vi "15-12-13 UHR-Fleezers Control (host) - 15.2.1UCB Darwin.vi"() -> ()   [LabVIEW 2014] (continued)
            n3419 = flat-sequence {
              frame #0 {
                # "stop only if saving"
                n3420 = local read "Saving..."() -> (w4631:bool)
                n3421 = And(x=w4631, y="TA Cancel Save?") -> (x .and. y?=w4630:bool)
                n3422 = local write "Stop Saving"(w4630) -> ()
              }
              frame #1 {
                n3423 = case shown="True" "TA Green Off?" {
                  frame False {
                  }
                  frame True {
                    w4634 = FALSE ("Fl. Triggered...")
                    n3424 = local write "Fl. Triggered..."(w4634) -> ()
                    n3425 = property on="Green Laser ON" class="Bool (strict)"("Val(Sgnl)"=w4634) -> ()  [unwired: 2 in, 2 out]
                  }
                }
              }
            }
            n3426 = local read "Time tether formed"() -> (w4625:timestamp)
            n3427 = Get Date/Time In Seconds() -> (seconds since 1Jan1904=w4626:timestamp)
            n3428 = Subtract(x=w4626, y=w4625) -> (x-y=w4624:dbl)
            n3429 = Number To Decimal String(number=w4624) -> (decimal integer string=w4621:string)  [unwired: 1 out]
            n3430 = local read "Messages"() -> (w4628:string)
            n3431 = call <vilib>:"Beep.vi"() -> ()  [unwired: 3 in, 9 out]
            n3432 = Concatenate Strings("Lost tether (" ("Message to add"), w4621, " s)." ("string")) -> (w4623:string)
            n3433 = local write "Tether"(FALSE ("Tether")) -> ()
            n3434 = call "Update messages.vi"("Message to add"=w4623, "Old message string"=w4628) -> ("New message string"=w4627:string)
            n3435 = local write "Messages"(w4627) -> ()
            n3436 = property on="Fl. Triggered..." class="Bool (strict)"("Val(Sgnl)"=w4619) -> ()  [unwired: 2 in, 2 out]
            n3437 = local write "Dip for Protein"(w4619) -> ()
            n3438 = property on="Trap Pos. FB ON" class="Bool (strict)"("Val(Sgnl)"=w4619) -> ()  [unwired: 2 in, 2 out]
            n3439 = property on="Trap Trig. Fl." class="Bool (strict)"("Val(Sgnl)"=w4619) -> ()  [unwired: 2 in, 2 out]
          }
        }
      }
    }
    n3440 = case "For triggering actions based on the trap position (e.g., turning the excitation laser on if trap under feedback moves so far)" shown="True" "Trap Trig. Fl." {
      tunnel: w4110 -> [_ w4507]
      tunnel: w4123 -> [_ w4506]
      tunnel: ["" ("t") w4505] -> w4131
      tunnel: w4115 -> [_ w4504]
      tunnel: [0 ("t") w4503] -> w4128
      tunnel: w4127 -> [_ w4502]
      tunnel: w4102 -> [_ w4501]
      tunnel: w4101 -> [_ w4500]
      frame False {
      }
      frame True {
        n3441 = case shown="\"Wait for trigger\"" w4506 {
          tunnel: w4507 -> [w4524 _ _ w4572]
          tunnel: [w4521 w4553 "" ("t") w4575] -> w4505
          tunnel: w4504 -> [_ _ _ w4563]
          tunnel: [w4520 w4550 0 ("t") w4564] -> w4503
          tunnel: w4502 -> [_ w4552 _ w4570]
          tunnel: w4501 -> [w4509 w4547 _ w4566]
          tunnel: w4500 -> [w4508 w4546 _ w4565]
          frame "Wait for trigger" {
            n3442 = local read "Trap Trig. (FPGA)"() -> (w4512:bool)
            n3443 = Subtract(x=w4524, y="Mean T1 Position\nto compare (nm)") -> (x-y=w4517:dbl[])
            n3444 = call <vilib>:"Std Deviation and Variance.vi"("X"=w4517) -> ("mean"=→"mean":dbl, "standard deviation"=→"standard\ndeviation":dbl)  [unwired: 1 in, 1 out]
            n3445 = Array Max & Min(array=w4517) -> (max value=→"max value":dbl, min value=→"min value":dbl)  [unwired: 2 out]
            n3446 = Greater?(x=w4517, y="Threshold (nm)") -> (0:w4527:bool[])
            n3447 = case shown="True" w4512 {
              tunnel: w4509 -> [_ w4533]
              tunnel: w4508 -> [_ w4532]
              tunnel: [FALSE ("TTrig?") w4531] -> w4515
              frame False {
              }
              frame True {
                n3448 = xnode "Read/Write Control"("FPGA VI Reference In"=w4533, "error in"=w4532) -> ("TTrig?"=w4531:bool)  [unwired: 2 out]
              }
            }
            n3449 = Or Array Elements(Boolean array=w4527) -> (logical OR=w4514:bool)
            n3450 = Select(t=w4515, s=w4512, f=w4514) -> (s? t:f=w4513:bool)
            n3451 = Not(x=w4512) -> (.not. x?=w4511:bool)
            n3452 = And(x=w4513, y=w4511) -> (x .and. y?=w4510:bool)
            n3453 = Select(t="Triggered", s=w4513, f="Wait for trigger") -> (s? t:f=w4521:string)
            n3454 = case shown="True" w4513 {
              tunnel: [0 0] -> w4520
              tunnel: w4509 -> [_ w4538]
              tunnel: w4508 -> [_ w4537]
              frame False {
                "Waiting" <- TRUE ("Waiting")
              }
              frame True {
                n3455 = xnode "Read/Write Control"("FPGA VI Reference In"=w4538, "error in"=w4537, "TTrig?"=FALSE) -> ()  [unwired: 2 out]
                n3456 = local read "Messages"() -> (w4541:string)
                n3457 = call <vilib>:"Beep.vi"() -> ()  [unwired: 12 in]
                n3458 = call "Update messages.vi"("Message to add"="Unwinding trigger.", "Old message string"=w4541) -> ("New message string"=w4542:string)
                n3459 = local write "Messages"(w4542) -> ()
                n3460 = local write "Waiting"(FALSE ("Waiting")) -> ()
                "Triggered" <- TRUE ("Triggered")
              }
            }
            n3461 = case "Only need to turn on laser if host triggered" shown="True" w4510 {
              frame False {
              }
              frame True {
                n3462 = property on="Green Laser ON" class="Bool (strict)"("Val(Sgnl)"=TRUE ("Value (Signaling)")) -> ()  [unwired: 2 in, 2 out]
              }
            }
          }
          frame "Triggered" {
            n3463 = local read "Trap Trig. (FPGA)"() -> (w4549:bool)
            n3464 = Increment(x=w4552) -> (x+1=w4550:i32)
            n3465 = Greater Or Equal?(x=w4550, y="Fl. ON time (n)") -> (x >= y?=w4548:bool)
            n3466 = Select(t="Wait for trigger", s=w4548, f="Triggered" ("t")) -> (s? t:f=w4553:string)
            n3467 = And(x=w4548, y=w4549) -> (x .and. y?=w4545:bool)
            n3468 = case shown="True" w4545 {
              tunnel: w4547 -> [_ w4557]
              tunnel: w4546 -> [_ w4556]
              frame False {
              }
              frame True {
                n3469 = xnode "Read/Write Control"("FPGA VI Reference In"=w4557, "error in"=w4556, "FPGA Trap Trig"=TRUE) -> ()  [unwired: 2 out]
              }
            }
            n3470 = case shown="True" w4548 {
              frame False {
              }
              frame True {
                w4559 = FALSE ("Value (Signaling)")
                n3471 = local write "Triggered"(w4559) -> ()
                n3472 = local write "Waiting"(TRUE ("Waiting")) -> ()
                n3473 = property on="Green Laser ON" class="Bool (strict)"("Val(Sgnl)"=w4559) -> ()  [unwired: 2 in, 2 out]
              }
            }
          }
          frame "Do nothing" {
          }
          frame "Initialize", Default {
            n3474 = Increment(x=w4570) -> (x+1=w4574:i32)
            n3475 = Select(t=1, s=w4563, f=w4574) -> (s? t:f=w4564:i32)
            n3476 = feedback #28(w4572) -> (w4578:dbl[])
            n3477 = Build Array (concatenate)(w4572, w4578) -> (w4571:dbl[])
            n3478 = Greater Or Equal?(x=w4564, y="Wait to get offset (n)") -> (x >= y?=w4567:bool)
            n3479 = Select(t=w4572, s=w4563, f=w4571) -> (s? t:f=w4573:dbl[])
            n3480 = feedback-in #28(w4573) -> ()
            n3481 = call-poly <vilib>:"Mean.vi"("X"=w4573) -> ("mean"=w4568:dbl)  [unwired: 1 out]
            n3482 = local write "Mean T1 Position\nto compare (nm)"(w4568) -> ()
            n3483 = case shown="True" w4563 {
              tunnel: w4566 -> [_ w4584]
              tunnel: w4565 -> [_ w4583]
              frame False {
              }
              frame True {
                w4580 = FALSE ("FPGA Trap Trig")
                n3484 = xnode "Read/Write Control"("FPGA VI Reference In"=w4584, "error in"=w4583, "FPGA Trap Trig"=w4580) -> ("FPGA VI Reference Out"=w4582:T24, "error out"=w4581:errorcluster)
                n3485 = xnode "Read/Write Control"("FPGA VI Reference In"=w4582, "error in"=w4581, "TTrig?"=w4580) -> ()  [unwired: 2 out]
              }
            }
            n3486 = Select(t="Wait for trigger", s=w4567, f="Initialize") -> (s? t:f=w4575:string)
            n3487 = case shown="True" w4567 {
              tunnel: w4568 -> [_ w4587]
              tunnel: w4566 -> [_ w4596]
              tunnel: w4565 -> [_ w4595]
              frame False {
                n3488 = local write "Waiting"(FALSE ("Waiting")) -> ()
                "Initializing" <- TRUE ("Initializing")
              }
              frame True {
                n3489 = local read "Threshold (nm)"() -> (w4599:dbl)
                n3490 = local read "AOM X Cal (nm/MHz)"() -> (w4598:dbl)
                n3491 = Add(x=w4587, y=w4599) -> (x+y=w4600:dbl)
                n3492 = Divide(x=w4600, y=w4598) -> (x/y=w4597:dbl)
                n3493 = call "IR AOM freq to word.vi"("Frequency In (MHz)"=w4597) -> ("Frequency Word Out (double)"=w4594:dbl)
                n3494 = local write "Initializing"(FALSE ("Initializing")) -> ()
                n3495 = local write "Waiting"(TRUE ("Waiting")) -> ()
                n3496 = To Quad Integer(1:w4594) -> (0:w4593:i64)
                n3497 = xnode "Read/Write Control"("FPGA VI Reference In"=w4596, "error in"=w4595, "FPGA TTrig Thresh"=w4593) -> ("FPGA VI Reference Out"=w4590:T24, "error out"=w4589:errorcluster)
                n3498 = xnode "Read/Write Control"("FPGA VI Reference In"=w4590, "error in"=w4589, "FPGA Trap Trig"=TRUE) -> ()  [unwired: 2 out]
              }
            }
          }
        }
      }
    }
    n3499 = feedback-in #26(w4131) -> ()
    n3500 = feedback-in #27(w4128) -> ()
    n3501 = xnode ("Read/Write Control")("FPGA VI Reference In"=w4270, "error in"=w4269) -> ("FPGA VI Reference Out"=w4113:T24, "error out"=w4112:errorcluster, "AI2 Y Sum Set 1"=w4342:i16, "AI2 Y Sum Set 2"=w4341:i16, "AI1 X Set 1"=w4177:fxp<+/-,16,1>, "AI1 X Set 2"=w4176:fxp<+/-,16,1>, "Trap Pos FB Int Signal"=→"Trap Pos FB Int Signal":fxp<+/-,24,9>, "Trap Pos FB Int-Norm Signal"=→"Trap Pos FB Int-Norm Signal":fxp<+/-,16,1>, "Trap Pos FB Action"=w4170:i64, "Scanning"=→"AOD Scanning":bool, "Scan I"=→"AOD Scan I":u64, "Scanning MCL"=w4344:bool, "Scan I (MCL)"=→"MCL Scan I":u64, "Green FB Sum"=w4286:i16, "Trap Pos FB Action"=w4100:i64, "TTrig Fin Thresh"=w4096:i64, "Red FB Intensity"=w4080:i16, "Blue Intensity"=w4075:i16)
    "MCL Scanning" <- w4344
    "Trap Pos FB Action" <- w4170
    n3502 = Divide(x=w4080, y=3276.7) -> (x/y=w4079:dbl)
    "Red laser intensity (V)" <- w4079
    n3503 = Divide(x=w4075, y=3276.7) -> (x/y=w4074:dbl)
    "Blue laser intensity (V)" <- w4074
    n3504 = Divide(x=w4286, y=3276.7) -> (x/y=w4078:dbl)
    "Green laser intensity (V)" <- w4078
    n3505 = local read "FB Trig Integrate"() -> (w4094:u32)
    n3506 = Divide(x=w4100, y=w4094) -> (x/y=w4093:dbl)
    "TTrig Sig (Int)" <- w4093
    n3507 = Bundle(w4078, w4079, w4074) -> (→"Fluorescence laser intensities plot":cluster{dbl, dbl, dbl})  [unwired: 1 in]
    n3508 = Divide(x=w4096, y=w4094) -> (x/y=w4091:dbl)
    "TTrig Fin Thresh (Int)" <- w4091
    n3509 = local read "AOM X Cal (nm/MHz)"() -> (w4099:dbl)
    n3510 = local read "AI2 (V)"() -> (w4343:cluster{"Set 1":dbl, "Set 2":dbl})
    n3511 = Bundle By Name(cluster=w4343, "Set 1"=w4342, "Set 2"=w4341) -> (w4339:cluster{"Set 1":dbl, "Set 2":dbl})
    n3512 = Divide(x=w4170, y=327.67) -> (x/y=→"Action (%)":dbl)
    n3513 = local read "Trap X (AI1)"() -> (w4190:T12)
    n3514 = call "IR AOM word double to freq.vi"("Frequency Word In (double)"=w4091) -> ("Frequency Out (MHz)"=w4090:dbl)
    n3515 = call "IR AOM word double to freq.vi"("Frequency Word In (double)"=w4093) -> ("Frequency Out (MHz)"=w4092:dbl)
    n3516 = Divide(x=w4339, y=3276.7) -> (x/y=w4338:cluster{"Set 1":dbl, "Set 2":dbl})
    n3517 = Multiply(x=w4092, y=w4099) -> (x*y=w4098:dbl)
    "TTrig Sig (nm)" <- w4098
    n3518 = Multiply(x=w4090, y=w4099) -> (x*y=w4097:dbl)
    "TTrig Fin Thresh (nm)" <- w4097
    n3519 = local write "AI2 (V)"(w4338) -> ()
    n3520 = Bundle(cluster=w4190, "Trap 1"=w4177, "Trap 2"=w4176) -> (→"Trap X (AI1)":T12)
    n3521 = Bundle(w4098, w4097) -> (→"TTrig":cluster{dbl, dbl})  [unwired: 1 in]
    n3522 = flat-sequence "To save data" {
      tunnel: [w5479] -> w4362
      tunnel: [w5480] -> w4361
      tunnel: w4315 -> [w5473]
      tunnel: w4118 -> [w5477]
      tunnel: ["Save Calibration"] -> w4335
      tunnel: w4332 -> [w5476]
      tunnel: [w5469] -> w4331
      tunnel: [w5466] -> w4330
      tunnel: [w5463] -> w4329
      tunnel: w4314 -> [w5465]
      tunnel: w4254 -> [w5459]
      tunnel: [w5459] -> w4253
      tunnel: [w5451] -> w4227
      tunnel: [w5454] -> w4158
      tunnel: [w5453] -> w4157
      tunnel: [w5447] -> w4008
      tunnel: w4362 -> [w5757]
      tunnel: w4361 -> [w5756]
      tunnel: w4159 -> [w5755]
      tunnel: w4335 -> [w5754]
      tunnel: w4331 -> [w5752]
      tunnel: w4330 -> [w5751]
      tunnel: w4329 -> [w5750]
      tunnel: w4235 -> [w5749]
      tunnel: w4262 -> [w5748]
      tunnel: w4253 -> [w5747]
      tunnel: w4227 -> [w5746]
      tunnel: w4015 -> [w5745]
      tunnel: w4060 -> [w5744]
      tunnel: w4158 -> [w5743]
      tunnel: w4157 -> [w5742]
      tunnel: w4156 -> [w5741]
      tunnel: w4082 -> [w5740]
      tunnel: w4006 -> [w5739]
      tunnel: w4008 -> [w5738]
      frame #0 {
        n3523 = Or(x="Start Saving", y="Start saving data + video") -> (x .or. y?=w5451:bool)
        n3524 = case shown="True" "Start saving data + video" {
          frame False {
          }
          frame True {
            n3525 = stacked-sequence {
              frame #0 {
                n3526 = local write "New Video File"(TRUE ("New Video File")) -> ()
              }
              frame #1 {
                n3527 = local write "Save Video"(TRUE ("Save Video")) -> ()
              }
            }
          }
        }
        n3528 = Or(x="Save N Sets", y=w5451) -> (x .or. y?=w5460:bool)
        n3529 = To Double Precision Float(number=w5476) -> (double precision float=w5470:dbl)
        n3530 = Build Array(w5460, "Save Calibration", w5473, w5465) -> (w5475:bool[])
        n3531 = Compound Arithmetic op=OR("Save Calibration", w5473, w5460, w5465) -> (w5478:bool)
        n3532 = Boolean Array To Number(Boolean array=w5475) -> (number=w5472:u32)
        n3533 = feedback #29(FALSE ("Save APD Data\nwith Trap Data")) -> (w5455:bool)
        n3534 = feedback #30(refnum<k0> refnum) -> (w5481:refnum<file>)
        n3535 = feedback #31(FALSE ("Save APD Data\nwith Trap Data")) -> (w5464:bool)
        n3536 = feedback #32(0) -> (w5483:i32)
        n3537 = feedback #33() -> (w5471:u32)  [unwired: 1 out]
        n3538 = feedback #34(refnum<k0> refnum) -> (w5448:refnum<file>)
        n3539 = feedback #35(refnum<k0> refnum) -> (w5457:refnum<file>)
        n3540 = feedback #36(refnum<k0> refnum) -> (w5467:refnum<file>)
        n3541 = case shown="True" w5478 {
          tunnel: [w5493 1] -> w5479
          tunnel: w5483 -> [w5495 _]
          tunnel: [w5494 w5528] -> w5480
          tunnel: w5481 -> [w5494 _]
          tunnel: w5477 -> [_ w5546]
          tunnel: w5470 -> [_ w5544]
          tunnel: w5472 -> [_ w5547]
          tunnel: [w5492 w5527] -> w5469
          tunnel: w5471 -> [w5492 _]
          tunnel: [w5491 w5525] -> w5466
          tunnel: w5467 -> [w5491 _]
          tunnel: [w5490 w5524] -> w5463
          tunnel: w5464 -> [w5490 _]
          tunnel: w5451 -> [_ w5522]
          tunnel: w5459 -> [_ w5521]
          tunnel: [w5489 w5513] -> w5453
          tunnel: w5457 -> [w5489 _]
          tunnel: [w5488 w5512] -> w5454
          tunnel: w5455 -> [w5488 _]
          tunnel: [w5487 w5496] -> w5447
          tunnel: w5448 -> [w5487 _]
          frame False {
            n3542 = Increment(x=w5495) -> (x+1=w5493:i32)
          }
          frame True {
            w5518 = FALSE ("Start Saving")
            w5523 = 9.0  # File Version
            w5530 = FALSE ("prepend array or string size? (T)")
            w5529 = T32."big-endian, network order" ("byte order (0:big-endian, network order)")
            # "Save trap position\ndata"
            n3543 = local read "BD 1 Frequency 1 (MHz)"() -> (w5543:dbl)
            n3544 = local read "BD 2 Frequency 1 (MHz)"() -> (w5542:dbl)
            n3545 = local read "BD 1 Frequency 2 (MHz)"() -> (w5541:dbl)
            n3546 = local read "BD 2 Frequency 2 (MHz)"() -> (w5540:dbl)
            n3547 = local read "BD 1 Frequency 3 (MHz)"() -> (w5539:dbl)
            n3548 = local read "BD 2 Frequency 3 (MHz)"() -> (w5538:dbl)
            n3549 = Array Size(array=w5521) -> (size(s)=w5520:i32)
            n3550 = To Double Precision Float(number=w5520) -> (double precision float=w5519:dbl)
            n3551 = local write "Save Calibration"(w5518) -> ()
            n3552 = local write "Start Saving"(w5518) -> ()
            n3553 = Build Array("Save APD Data\nwith Trap Data", "Save Trap Pos. Data") -> (w5515:bool[])
            n3554 = Boolean Array To Number(Boolean array=w5515) -> (number=w5514:u32)
            n3555 = Build Array(w5543, w5542, w5541, w5540, w5539, w5538) -> (w5537:dbl[])
            n3556 = case shown="2" w5547 {
              tunnel: w5546 -> [w5635 w5662 w5678 w5716]
              tunnel: w5519 -> [w5640 w5669 w5698 w5735]
              tunnel: w5544 -> [w5639 w5668 w5697 w5734]
              tunnel: [w5636 w5664 w5689 w5726] -> w5535
              tunnel: [w5627 "Cal sets to save" w5679 w5717] -> w5527
              tunnel: w5537 -> [w5637 w5665 w5691 w5728]
              tunnel: "Save APD Data\nwith Trap Data" -> [w5634 w5651 w5675 w5714]
              tunnel: [w5634 w5649 w5675 w5714] -> w5524
              tunnel: w5523 -> [w5630 w5658 w5673 w5712]
              tunnel: w5522 -> [w5629 _ _ _]
              tunnel: [w5620 w5657 w5672 w5702] -> w5512
              tunnel: "Save Trap Pos. Data" -> [w5620 w5656 w5672 w5702]
              tunnel: w5514 -> [w5619 w5655 w5671 w5701]
              frame 1, Default {
                # "timeseries"
                n3557 = case shown="False" "Profile" {
                  tunnel: [w5643 w5647] -> w5624
                  tunnel: [w5643 w5646] -> w5623
                  tunnel: [w5643 w5645] -> w5622
                  tunnel: [w5643 w5644] -> w5621
                  frame False {
                    w5643 = 0.0 ("f")
                  }
                  frame True {
                    n3558 = local read "Current Position"() -> (w5648:cluster{dbl, dbl, dbl})
                    n3559 = local read "Y change (mm)"() -> (w5644:dbl)
                    n3560 = Unbundle(w5648) -> (w5647:dbl, w5646:dbl, w5645:dbl)
                  }
                }
                n3561 = local read "Save ave N"() -> (w5642:dbl)
                n3562 = Multiply(x=w5642, y=w5635) -> (x*y=w5641:dbl)
                n3563 = To Double Precision Float(number=w5619) -> (double precision float=w5633:dbl)
                n3564 = Build Array(w5630, w5635, w5641, w5640, w5639, 0.0 ("f")) -> (w5638:dbl[])
                n3565 = Build Array(w5633, w5624, w5623, w5622, w5621) -> (w5631:dbl[])
                n3566 = Select(t=u32 4000000000, s=w5629, f="N sets to save") -> (s? t:f=w5627:u32)
                n3567 = Build Array (concatenate)(w5638, w5637, w5631) -> (w5636:dbl[])
              }
              frame 2 {
                w5660 = 0.0 ("f")
                w5650 = FALSE ("Save APD Data\nwith Trap Data")
                # "For diagnostics save trap position\ndata during cal"
                # "calibration"
                n3568 = Boolean To (0,1)(Boolean=w5650) -> (0, 1=w5654:i16)
                n3569 = Select(t=w5651, s="Save trap pos with cal", f=w5650) -> (s? t:f=w5649:bool)
                n3570 = Select(t=w5656, s="Save trap pos with cal", f=w5650) -> (s? t:f=w5657:bool)
                n3571 = Select(t=w5655, s="Save trap pos with cal", f=w5654) -> (s? t:f=w5653:u32)
                n3572 = To Double Precision Float(number=w5653) -> (double precision float=w5661:dbl)
                n3573 = Build Array(w5658, w5662, w5662, w5669, w5668, 1.0 ("t")) -> (w5666:dbl[])
                n3574 = Build Array(w5661, w5660, w5660, w5660, w5660) -> (w5659:dbl[])
                n3575 = Build Array (concatenate)(w5666, w5665, w5659) -> (w5664:dbl[])
                "Calibrating Trap..." <- TRUE ("Calibrating...")
              }
              frame 4 {
                w5676 = 0.0 ("f")
                # "scan dir (x/y = 0/1)"
                # "cycles/step"
                # "n scans (f/b)"
                # "steps"
                # "freq. range"
                # "AOD raster scan"
                n3576 = local read "Number of F/B Scans (AOD)"() -> (w5683:u16)
                n3577 = local read "Cycles/step (AOD)"() -> (w5685:u64)
                n3578 = local read "Scan Range (MHz)"() -> (w5688:dbl)
                n3579 = local read "Scan steps (AOD)"() -> (w5687:u64)
                n3580 = local read "Scan BD"() -> (w5695:bool)
                n3581 = local read "Save ave N"() -> (w5700:dbl)
                n3582 = Boolean To (0,1)(Boolean=w5695) -> (0, 1=w5694:i16)
                n3583 = To Double Precision Float(number=w5683) -> (double precision float=w5682:dbl)
                n3584 = To Double Precision Float(number=w5687) -> (double precision float=w5686:dbl)
                n3585 = To Double Precision Float(number=w5685) -> (double precision float=w5684:dbl)
                n3586 = To Double Precision Float(number=w5694) -> (double precision float=w5693:dbl)
                n3587 = Multiply(x=w5700, y=w5678) -> (x*y=w5699:dbl)
                n3588 = To Double Precision Float(number=w5671) -> (double precision float=w5677:dbl)
                n3589 = Build Array(w5677, w5676, w5676, w5676, w5676) -> (w5674:dbl[])
                n3590 = local read "N sets should be saved"() -> (w5680:dbl)
                n3591 = Build Array(w5693, w5688, w5686, w5684, w5682) -> (w5690:dbl[])
                n3592 = Build Array(w5673, w5678, w5699, w5698, w5697, 2.0 ("t")) -> (w5692:dbl[])
                n3593 = Round Toward +Infinity(x=w5680) -> (ceil(x): smallest int >= x=w5681:dbl)
                n3594 = Build Array (concatenate)(w5692, w5691, w5674, w5690) -> (w5689:dbl[])
                n3595 = To Unsigned Long Integer(number=w5681) -> (unsigned 32bit integer=w5679:u32)
              }
              frame 8 {
                w5709 = 0.0 ("f")
                # "MCL raster scan"
                n3596 = local read "Number of scans (MCL)"() -> (w5704:u64)
                n3597 = local read "Scan lines (y)"() -> (w5703:u64)
                n3598 = local read "2D or 1D Scan"() -> (w5706:bool)
                n3599 = local read "Scan Range (V)\n(of steps)"() -> (w5725:dbl)
                n3600 = local read "Fast Scan Dir"() -> (w5732:bool)
                n3601 = local read "Cycles/step (MCL)"() -> (w5722:u64)
                n3602 = local read "Scan steps (MCL)"() -> (w5724:u64)
                n3603 = Select(t=w5703, s=w5706, f=w5704) -> (s? t:f=w5705:u64)
                n3604 = Boolean To (0,1)(Boolean=w5706) -> (0, 1=w5708:i16)
                n3605 = local read "Save ave N"() -> (w5737:dbl)
                n3606 = local read "Initial X"() -> (w5711:dbl)
                n3607 = local read "Initial Y"() -> (w5710:dbl)
                n3608 = To Double Precision Float(number=w5708) -> (double precision float=w5707:dbl)
                n3609 = Boolean To (0,1)(Boolean=w5732) -> (0, 1=w5731:i16)
                n3610 = To Double Precision Float(number=w5705) -> (double precision float=w5720:dbl)
                n3611 = To Double Precision Float(number=w5724) -> (double precision float=w5723:dbl)
                n3612 = To Double Precision Float(number=w5722) -> (double precision float=w5721:dbl)
                n3613 = To Double Precision Float(number=w5731) -> (double precision float=w5730:dbl)
                n3614 = Multiply(x=w5737, y=w5716) -> (x*y=w5736:dbl)
                n3615 = To Double Precision Float(number=w5701) -> (double precision float=w5715:dbl)
                n3616 = local read "N sets should be saved (MCL)"() -> (w5718:dbl)
                n3617 = Build Array(w5715, w5707, w5709, w5709, w5709) -> (w5713:dbl[])
                n3618 = Build Array(w5730, w5725, w5723, w5721, w5720, w5711, w5710) -> (w5727:dbl[])
                n3619 = Build Array(w5712, w5716, w5736, w5735, w5734, 3.0 ("t")) -> (w5729:dbl[])
                n3620 = Round Toward +Infinity(x=w5718) -> (ceil(x): smallest int >= x=w5719:dbl)
                n3621 = Build Array (concatenate)(w5729, w5728, w5713, w5727) -> (w5726:dbl[])
                n3622 = To Unsigned Long Integer(number=w5719) -> (unsigned 32bit integer=w5717:u32)
              }
            }
            n3623 = local read "Index"() -> (w5552:dbl)
            n3624 = call "Create new save file.vi"("Insert"="", "Ext"=".dat", "Index In"=w5552) -> ("Path Out"=w5498:path, "Index Out"=w5526:dbl)
            n3625 = local write "Save file name"(w5498) -> ()
            n3626 = local write "Index"(w5526) -> ()
            n3627 = local write "Save index"(w5526) -> ()
            n3628 = case shown="True" "Save Event Log?" {
              tunnel: w5498 -> [_ w5560]
              tunnel: [refnum<k0> refnum w5559] -> w5496
              frame False {
              }
              frame True {
                (unwired) FALSE ("prepend array or string size? (T)")
                n3629 = Path To String(path=w5560) -> (string=w5571:string)
                n3630 = String Length(string=w5571) -> (length=w5570:i32)
                n3631 = Subtract(x=w5570, y=4) -> (x-y=w5568:i32)
                n3632 = String Subset(string=w5571, length (rest)=w5568) -> (substring=w5567:string)  [unwired: 1 out]
                n3633 = Concatenate Strings(w5567, "_log.txt" ("string")) -> (w5565:string)
                n3634 = String To Path(string=w5565) -> (path=w5561:path)
                n3635 = Open/Create/Replace File(file path (use dialog)=w5561, operation (0:open)=T33."create", access (0:read/write)=enum16{"read/write", "read-only", "write-only"}."write-only") -> (refnum out=w5562:refnum<file>)  [unwired: 1 in, 4 out]
                n3636 = Deny Access(7:w5562) -> (3:w5559:refnum<file>)  [unwired: 1 in, 2 out]
                n3637 = call "write to event log.vi"("log file ref"=w5559, "time"=0.0, "input string"="start log") -> ()  [unwired: 8 in]
              }
            }
            "log file ref" <- w5496
            n3638 = Array Size(array=w5535) -> (size(s)=w5536:i32)
            n3639 = Open/Create/Replace File(file path (use dialog)=w5498, operation (0:open)=T33."create", access (0:read/write)=enum16{"read/write", "read-only", "write-only"}."write-only") -> (refnum out=w5549:refnum<file>)  [unwired: 1 in, 4 out]
            n3640 = local write "Saving..."(TRUE ("Saving...")) -> ()
            n3641 = To Double Precision Float(number=w5536) -> (double precision float=w5534:dbl)
            n3642 = String Length(string="Comment (data description)") -> (length=w5533:i32)
            n3643 = To Double Precision Float(number=w5533) -> (double precision float=w5532:dbl)
            n3644 = Deny Access(7:w5549) -> (3:w5548:refnum<file>)  [unwired: 1 in, 2 out]
            n3645 = Build Array (concatenate)(w5534, w5535, w5532) -> (w5508:dbl[])
            n3646 = case "If fluorescence data to be saved" shown="True" w5524 {
              tunnel: w5498 -> [_ w5618]
              tunnel: [refnum<k0> refnum w5598] -> w5525
              frame False {
              }
              frame True {
                w5597 = 0.0
                n3647 = local read "APD Integration Time (s)"() -> (w5603:dbl)
                n3648 = local read "N APD Samp/step"() -> (w5596:dbl)
                n3649 = local read "Number of APDs"() -> (w5595:u8)
                n3650 = Path To String(path=w5618) -> (string=w5617:string)
                n3651 = String Length(string=w5617) -> (length=w5616:i32)
                n3652 = Subtract(x=w5616, y=4) -> (x-y=w5614:i32)
                n3653 = String Subset(string=w5617, length (rest)=w5614) -> (substring=w5613:string)  [unwired: 1 out]
                n3654 = Build Array(w5603, w5596, w5595, w5597, w5597, w5597, w5597, w5597) -> (w5600:dbl[])
                n3655 = Concatenate Strings(w5613, "_fl.dat" ("string")) -> (w5611:string)
                n3656 = Array Size(array=w5600) -> (size(s)=w5602:i32)
                n3657 = String To Path(string=w5611) -> (path=w5607:path)
                n3658 = Open/Create/Replace File(file path (use dialog)=w5607, operation (0:open)=T33."create", access (0:read/write)=enum16{"read/write", "read-only", "write-only"}."write-only") -> (refnum out=w5608:refnum<file>)  [unwired: 1 in, 4 out]
                n3659 = Deny Access(7:w5608) -> (3:w5604:refnum<file>)  [unwired: 1 in, 2 out]
                n3660 = To Double Precision Float(number=w5602) -> (double precision float=w5601:dbl)
                n3661 = Build Array (concatenate)(w5601, w5600) -> (w5599:dbl[])
                n3662 = Write to Binary File(file (use dialog)=w5604, data=w5599, 5:FALSE ("prepend array or string size? (T)"), 9:T32."big-endian, network order" ("byte order (0:big-endian, network order)")) -> (refnum out=w5598:refnum<file>)  [unwired: 1 in, 3 out]
              }
            }
            n3663 = case shown="True" w5512 {
              tunnel: w5498 -> [_ w5579]
              tunnel: [refnum<k0> refnum w5578] -> w5513
              frame False {
              }
              frame True {
                w5574 = 0.0 ("element")
                n3664 = Path To String(path=w5579) -> (string=w5593:string)
                n3665 = Build Array(w5574, w5574, w5574, w5574, w5574, w5574, w5574, w5574) -> (w5575:dbl[])
                n3666 = String Length(string=w5593) -> (length=w5592:i32)
                n3667 = Subtract(x=w5592, y=4) -> (x-y=w5590:i32)
                n3668 = Array Size(array=w5575) -> (size(s)=w5577:i32)
                n3669 = String Subset(string=w5593, length (rest)=w5590) -> (substring=w5589:string)  [unwired: 1 out]
                n3670 = To Double Precision Float(number=w5577) -> (double precision float=w5576:dbl)
                n3671 = Concatenate Strings(w5589, "_pos.dat" ("string")) -> (w5587:string)
                n3672 = Build Array (concatenate)(w5576, w5575) -> (w5573:dbl[])
                n3673 = String To Path(string=w5587) -> (path=w5583:path)
                n3674 = Open/Create/Replace File(file path (use dialog)=w5583, operation (0:open)=T33."create", access (0:read/write)=enum16{"read/write", "read-only", "write-only"}."write-only") -> (refnum out=w5584:refnum<file>)  [unwired: 1 in, 4 out]
                n3675 = Deny Access(7:w5584) -> (3:w5580:refnum<file>)  [unwired: 1 in, 2 out]
                n3676 = Write to Binary File(file (use dialog)=w5580, data=w5573, 5:FALSE ("prepend array or string size? (T)"), 9:T32."big-endian, network order" ("byte order (0:big-endian, network order)")) -> (refnum out=w5578:refnum<file>)  [unwired: 1 in, 3 out]
              }
            }
            n3677 = Write to Binary File(file (use dialog)=w5548, data=w5508, 5:w5530, 9:w5529) -> (refnum out=w5531:refnum<file>)  [unwired: 1 in, 3 out]
            n3678 = Write to Binary File(file (use dialog)=w5531, data="Comment (data description)", 5:w5530, 9:w5529) -> (refnum out=w5528:refnum<file>)  [unwired: 1 in, 3 out]
            n3679 = local read "connection reference"() -> (w5510:T19)
            n3680 = Bundle("Comment (data description)"="Comment (data description)", "Channel 1 Buffer"="Channel 1 Buffer", "Channel 2 Buffer"="Channel 2 Buffer", "Channel 3 Buffer"="Channel 3 Buffer", "Title"="Title", "DNA Construct"="DNA Construct", "Bead diameter"="Bead diameter", "Name"="Name") -> (w5499:T55)  [unwired: 1 in]
            n3681 = call "MattFileCreator-v9.vi"("Comments"=w5499, "Input Array"=w5508, "File path"=w5498, "table"="labview", "connection reference"=w5510) -> ("connection reference out"=w5509:T19)  [unwired: 5 in, 1 out]
            n3682 = local write "connection reference"(w5509) -> ()
          }
        }
        n3683 = feedback-in #29(w5454) -> ()
        n3684 = feedback-in #30(w5480) -> ()
        n3685 = feedback-in #31(w5463) -> ()
        n3686 = feedback-in #32(w5479) -> ()
        n3687 = feedback-in #33(w5469) -> ()
        n3688 = feedback-in #34(w5447) -> ()
        n3689 = feedback-in #35(w5453) -> ()
        n3690 = feedback-in #36(w5466) -> ()
      }
      frame #1 {
        n3691 = local read "Saving..."() -> (w5753:bool)
        n3692 = case shown="True" w5753 {
          tunnel: w5757 -> [_ w5771]
          tunnel: w5756 -> [_ w5785]
          tunnel: w5755 -> [_ w5781]
          tunnel: w5754 -> [_ w5780]
          tunnel: w5752 -> [_ w5779]
          tunnel: w5751 -> [_ w5774]
          tunnel: w5750 -> [_ w5773]
          tunnel: w5749 -> [_ w5772]
          tunnel: w5748 -> [_ w5770]
          tunnel: w5747 -> [_ w5768]
          tunnel: w5746 -> [_ w5767]
          tunnel: w5745 -> [_ w5766]
          tunnel: w5744 -> [_ w5765]
          tunnel: w5743 -> [_ w5764]
          tunnel: w5742 -> [_ w5763]
          tunnel: w5741 -> [_ w5762]
          tunnel: w5740 -> [_ w5761]
          tunnel: w5739 -> [_ w5759]
          tunnel: w5738 -> [_ w5758]
          frame False {
          }
          frame True {
            n3693 = case shown="True" "Stop saving data + video" {
              frame False {
              }
              frame True {
                n3694 = local write "Save Video"(FALSE ("Save Video")) -> ()
              }
            }
            n3695 = Multiply(x=w5771, y=w5770) -> (x*y=→"Time (s)":dbl)
            n3696 = Less Or Equal?(x=w5771, y=w5779) -> (x <= y?=w5783:bool)
            n3697 = Compound Arithmetic op=OR("Stop Saving", "Abort save 2", "Stop saving data + video") -> (w5775:bool)
            n3698 = Not(x=w5775) -> (.not. x?=w5784:bool)
            n3699 = And(x=w5783, y=w5784) -> (x .and. y?=w5782:bool)
            n3700 = case shown="False" w5782 {
              tunnel: w5785 -> [w5795 w5894]
              tunnel: [0.0 w5897] -> w5778
              tunnel: w5771 -> [_ w5895]
              tunnel: w5779 -> [_ w5896]
              tunnel: w5781 -> [_ w5891]
              tunnel: w5780 -> [_ _]
              tunnel: w5774 -> [w5793 w5884]
              tunnel: w5773 -> [w5792 w5885]
              tunnel: w5772 -> [_ w5883]
              tunnel: w5768 -> [_ w5882]
              tunnel: w5767 -> [_ w5800]
              tunnel: w5766 -> [_ w5875]
              tunnel: w5765 -> [_ w5822]
              tunnel: w5764 -> [w5789 w5839]
              tunnel: w5763 -> [w5790 w5838]
              tunnel: w5762 -> [_ w5835]
              tunnel: w5761 -> [_ w5833]
              tunnel: w5759 -> [_ w5799]
              tunnel: w5758 -> [w5788 _]
              frame False {
                w5791 = FALSE
                n3701 = Close File(refnum=w5795) -> ()  [unwired: 1 in, 2 out]
                n3702 = case shown="True" w5792 {
                  tunnel: w5793 -> [_ w5798]
                  frame False {
                  }
                  frame True {
                    n3703 = Close File(refnum=w5798) -> ()  [unwired: 1 in, 2 out]
                  }
                }
                n3704 = case shown="True" w5789 {
                  tunnel: w5790 -> [_ w5797]
                  frame False {
                  }
                  frame True {
                    n3705 = Close File(refnum=w5797) -> ()  [unwired: 1 in, 2 out]
                  }
                }
                n3706 = local read "Save Event Log?"() -> (w5787:bool)
                n3707 = case shown="True" w5787 {
                  tunnel: w5788 -> [_ w5796]
                  frame False {
                  }
                  frame True {
                    n3708 = Close File(refnum=w5796) -> ()  [unwired: 1 in, 2 out]
                  }
                }
                n3709 = local write "Raster Scanning..."(w5791) -> ()
                n3710 = local write "Calibrating Trap..."(w5791) -> ()
                n3711 = call <vilib>:"Beep.vi"() -> ()  [unwired: 3 in, 9 out]
                n3712 = local write "Stop Saving"(w5791) -> ()
                "Saving..." <- w5791
              }
              frame True {
                n3713 = local read "Calibrating Trap..."() -> (w5886:bool)
                n3714 = case "Write fl. data" shown="True" w5885 {
                  tunnel: w5884 -> [_ w5920]
                  tunnel: w5883 -> [_ w5919]
                  frame False {
                  }
                  frame True {
                    n3715 = Write to Binary File(file (use dialog)=w5920, data=w5919, 5:FALSE ("prepend array or string size? (T)"), 9:T32."big-endian, network order" ("byte order (0:big-endian, network order)")) -> ()  [unwired: 1 in, 4 out]
                  }
                }
                n3716 = Greater?(x="Save ave N", y=1.0) -> (0:w5889:bool)
                n3717 = Not(x=w5886) -> (.not. x?=w5888:bool)
                n3718 = And(x=w5888, y=w5889) -> (x .and. y?=w5836:bool)
                n3719 = case shown="True" w5836 {
                  tunnel: w5835 -> [w5900 w5911]
                  tunnel: [w5900 w5903] -> w5834
                  tunnel: "Save ave N" -> [_ w5904]
                  frame False {
                  }
                  frame True {
                    w5901 = 2 ("dimension size")
                    n3720 = Array Size(array=w5911) -> (size(s)=w5905:i32)
                    n3721 = Divide(x=w5905, y=w5901) -> (x/y=w5909:dbl)
                    n3722 = Reshape Array(w5911, w5909, w5901) -> (w5910:u64[][])
                    n3723 = Transpose 2D Array(2D array=w5910) -> (transposed array=w5908:u64[][])
                    n3724 = for {
                      tunnel: w5908 -> [w5913] mode=indexing
                      tunnel: [w5912] -> w5902 mode=indexing
                      tunnel: w5904 -> [w5914]
                      workers-P: _ -> [_]
                      n3725 = call "downsample 1D array - U64.vi"("Ave N"=w5914, "Array In"=w5913) -> ("Array Out"=w5912:u64[])  [unwired: 1 in]
                    }
                    n3726 = Transpose 2D Array(2D array=w5902) -> (transposed array=w5907:u64[][])
                    n3727 = Divide(x=w5905, y=w5904) -> (x/y=w5906:dbl)
                    n3728 = Reshape Array(w5907, w5906) -> (w5903:u64[])
                  }
                }
                n3729 = case shown="True" w5836 {
                  tunnel: w5891 -> [w5923 w5935]
                  tunnel: [w5923 w5927] -> w5887
                  tunnel: "Save ave N" -> [_ w5928]
                  tunnel: w5882 -> [_ w5926]
                  frame False {
                  }
                  frame True {
                    n3730 = Array Size(array=w5935) -> (size(s)=w5929:i32)
                    n3731 = Array Size(array=w5926) -> (size(s)=w5925:i32)
                    n3732 = Divide(x=w5929, y=w5925) -> (x/y=w5933:dbl)
                    n3733 = Reshape Array(w5935, w5933, w5925) -> (w5934:i16[][])
                    n3734 = Transpose 2D Array(2D array=w5934) -> (transposed array=w5932:i16[][])
                    n3735 = for {
                      tunnel: w5932 -> [w5938] mode=indexing
                      tunnel: [w5937] -> w5924 mode=indexing
                      tunnel: w5928 -> [w5936]
                      workers-P: _ -> [_]
                      n3736 = call "downsample 1D array - I16.vi"("Ave N"=w5936, "Array In"=w5938) -> ("Array Out"=w5937:i16[])  [unwired: 1 out]
                    }
                    n3737 = Transpose 2D Array(2D array=w5924) -> (transposed array=w5931:i16[][])
                    n3738 = Divide(x=w5929, y=w5928) -> (x/y=w5930:dbl)
                    n3739 = Reshape Array(w5931, w5930) -> (w5927:i16[])
                  }
                }
                n3740 = Index Array(array=w5822, index=2) -> (element=w5823:waveform(dbl))
                n3741 = Index Array(array=w5822, index=1) -> (element=w5856:waveform(dbl))
                n3742 = Index Array(array=w5822, index=0) -> (element=w5858:waveform(dbl))
                n3743 = Unbundle By Name(w5823) -> ("Y"=w5825:dbl[])
                n3744 = Unbundle By Name(w5856) -> ("Y"=w5860:dbl[])
                n3745 = Unbundle By Name(w5858) -> ("Y"=w5868:dbl[])
                n3746 = case "Write trap pos. data" shown="True" w5839 {
                  tunnel: w5838 -> [_ w5916]
                  tunnel: w5834 -> [_ w5915]
                  frame False {
                  }
                  frame True {
                    n3747 = Write to Binary File(file (use dialog)=w5916, data=w5915, 5:FALSE ("prepend array or string size? (T)"), 9:T32."big-endian, network order" ("byte order (0:big-endian, network order)")) -> ()  [unwired: 1 in, 4 out]
                  }
                }
                n3748 = Write to Binary File(file (use dialog)=w5894, data=w5887, 5:FALSE ("prepend array or string size? (T)"), 9:T32."big-endian, network order" ("byte order (0:big-endian, network order)")) -> ()  [unwired: 1 in, 4 out]
                n3749 = feedback #37(w5825) -> (w5826:dbl[])
                n3750 = Build Array (concatenate)(w5826, w5825) -> (w5821:dbl[])
                n3751 = Select(t=w5825, s=w5800, f=w5821) -> (s? t:f=w5811:dbl[])
                n3752 = feedback-in #37(w5811) -> ()
                n3753 = feedback #38(w5860) -> (w5862:dbl[])
                n3754 = Build Array (concatenate)(w5862, w5860) -> (w5861:dbl[])
                n3755 = Select(t=w5860, s=w5800, f=w5861) -> (s? t:f=w5850:dbl[])
                n3756 = feedback-in #38(w5850) -> ()
                n3757 = feedback #39(w5868) -> (w5881:dbl[])
                n3758 = Build Array (concatenate)(w5881, w5868) -> (w5880:dbl[])
                n3759 = Select(t=w5868, s=w5800, f=w5880) -> (s? t:f=w5855:dbl[])
                n3760 = feedback-in #39(w5855) -> ()
                n3761 = Divide(x=w5895, y=w5896) -> (x/y=w5898:dbl)
                n3762 = Multiply(x=w5898, y=100.0) -> (x*y=w5897:dbl)
                n3763 = Build Array(w5855, w5850, w5811) -> (→"Saved APD":dbl[][])
                n3764 = Array Size(array=w5855) -> (size(s)=w5873:i32)
                n3765 = Unbundle By Name(w5875) -> ("Y"=w5879:dbl[])
                n3766 = Subtract(x=w5873, y="N pts to average") -> (x-y=w5808:i32)
                n3767 = Multiply(x="N pts to average", y=u16 2) -> (x*y=w5851:u16)
                n3768 = Subtract(x=w5873, y=w5851) -> (x-y=w5809:i32)
                n3769 = feedback #40(w5879) -> (w5878:dbl[])
                n3770 = Build Array (concatenate)(w5878, w5879) -> (w5877:dbl[])
                n3771 = Select(t=w5879, s=w5800, f=w5877) -> (s? t:f=w5876:dbl[])
                "Trap Delta Graph" <- w5876
                n3772 = feedback-in #40(w5876) -> ()
                n3773 = Array Subset(array=w5855, index=w5808, length="N pts to average") -> (w5872:dbl[])
                n3774 = Array Subset(array=w5855, index=w5809, length="N pts to average") -> (w5871:dbl[])
                n3775 = Array Subset(array=w5850, index=w5808, length="N pts to average") -> (w5853:dbl[])
                n3776 = Array Subset(array=w5850, index=w5809, length="N pts to average") -> (w5852:dbl[])
                n3777 = Array Subset(array=w5811, index=w5808, length="N pts to average") -> (w5820:dbl[])
                n3778 = Array Subset(array=w5811, index=w5809, length="N pts to average") -> (w5819:dbl[])
                n3779 = Index Array(array=w5833, index=0) -> (element=w5831:waveform(dbl))
                n3780 = call-poly <vilib>:"Mean.vi"("X"=w5872) -> ("mean"=w5870:dbl)  [unwired: 1 out]
                n3781 = call-poly <vilib>:"Mean.vi"("X"=w5853) -> ("mean"=w5849:dbl)  [unwired: 1 out]
                n3782 = call-poly <vilib>:"Mean.vi"("X"=w5871) -> ("mean"=w5869:dbl)  [unwired: 1 out]
                n3783 = call-poly <vilib>:"Mean.vi"("X"=w5852) -> ("mean"=w5848:dbl)  [unwired: 1 out]
                n3784 = call-poly <vilib>:"Mean.vi"("X"=w5820) -> ("mean"=w5818:dbl)  [unwired: 1 out]
                n3785 = call-poly <vilib>:"Mean.vi"("X"=w5819) -> ("mean"=w5817:dbl)  [unwired: 1 out]
                n3786 = Unbundle By Name(w5831) -> ("Y"=w5829:dbl[])
                n3787 = Subtract(x=w5849, y=w5848) -> (x-y=w5840:dbl)
                "Delta Fl. 2" <- w5840
                n3788 = Subtract(x=w5818, y=w5817) -> (x-y=w5812:dbl)
                "Delta Fl. 3" <- w5812
                n3789 = Subtract(x=w5870, y=w5869) -> (x-y=w5867:dbl)
                "Delta Fl. 1" <- w5867
                n3790 = feedback #41(w5829) -> (w5828:dbl[])
                n3791 = Build Array (concatenate)(w5828, w5829) -> (w5830:dbl[])
                n3792 = Initialize Array(w5867, 1 ("dimension size")) -> (w5864:dbl[])
                n3793 = Initialize Array(w5840, 1 ("dimension size")) -> (w5845:dbl[])
                n3794 = Initialize Array(w5812, 1 ("dimension size")) -> (w5814:dbl[])
                n3795 = Select(t=w5829, s=w5800, f=w5830) -> (s? t:f=w5827:dbl[])
                "Saved trap pos" <- w5827
                n3796 = feedback-in #41(w5827) -> ()
                n3797 = feedback #42(w5864) -> (w5865:dbl[])
                n3798 = Build Array (concatenate)(w5865, w5864) -> (w5863:dbl[])
                n3799 = feedback #43(w5845) -> (w5846:dbl[])
                n3800 = feedback #44(w5814) -> (w5815:dbl[])
                n3801 = Build Array (concatenate)(w5846, w5845) -> (w5844:dbl[])
                n3802 = Build Array (concatenate)(w5815, w5814) -> (w5813:dbl[])
                n3803 = Select(t=w5864, s=w5800, f=w5863) -> (s? t:f=w5843:dbl[])
                n3804 = feedback-in #42(w5843) -> ()
                n3805 = Select(t=w5845, s=w5800, f=w5844) -> (s? t:f=w5842:dbl[])
                n3806 = feedback-in #43(w5842) -> ()
                n3807 = Select(t=w5814, s=w5800, f=w5813) -> (s? t:f=w5807:dbl[])
                n3808 = feedback-in #44(w5807) -> ()
                n3809 = Build Array(w5843, w5842, w5807) -> (→"Save APD Deriv":dbl[][])
                n3810 = Index Array(array=w5799, index=15) -> (element=w5805:waveform(dbl))
                n3811 = Unbundle By Name(w5805) -> ("Y"=w5803:dbl[])
                n3812 = feedback #45(w5803) -> (w5802:dbl[])
                n3813 = Build Array (concatenate)(w5802, w5803) -> (w5804:dbl[])
                n3814 = Select(t=w5803, s=w5800, f=w5804) -> (s? t:f=w5801:dbl[])
                "Amp current" <- w5801
                n3815 = feedback-in #45(w5801) -> ()
              }
            }
            "Progress" <- w5778
            "Progress 2" <- w5778
          }
        }
      }
    }
    n3816 = local read "wait to reset values"() -> (w4346:bool)
    n3817 = Not(x=w4344) -> (.not. x?=w4347:bool)
    n3818 = And(x=w4347, y=w4346) -> (x .and. y?=w4348:bool)
    n3819 = case "Part of MCL raster scanning: returns to initial positions after scan done" shown="True" w4348 {
      tunnel: w4113 -> [w5268 w5275]
      tunnel: [w5268 w5274] -> w4350
      tunnel: w4112 -> [w5267 w5273]
      tunnel: [w5267 w5272] -> w4345
      frame False {
      }
      frame True {
        w5283 = 10.0 ("y")
        w5282 = 32767.0 ("y")
        # "to return scan values\nafter a synchronous \nAOM scan"
        n3820 = local read "AO2"() -> (w5276:dbl)
        n3821 = local read "AO1"() -> (w5277:dbl)
        n3822 = local write "wait to reset values"(FALSE ("wait to reset values")) -> ()
        n3823 = Multiply(x=w5277, y=w5282) -> (x*y=w5279:dbl)
        n3824 = Multiply(x=w5276, y=w5282) -> (x*y=w5281:dbl)
        n3825 = Divide(x=w5279, y=w5283) -> (x/y=w5278:dbl)
        n3826 = Divide(x=w5281, y=w5283) -> (x/y=w5280:dbl)
        n3827 = To Word Integer(number=w5278) -> (16bit integer=w5284:i16)
        n3828 = To Word Integer(number=w5280) -> (16bit integer=w5285:i16)
        n3829 = local read "Total Counts (ticks)"() -> (w5269:u16)
        n3830 = xnode "Read/Write Control"("FPGA VI Reference In"=w5275, "error in"=w5273, "AO1"=w5284, "AO2"=w5285, "MCL count"=w5269) -> ("FPGA VI Reference Out"=w5274:T24, "error out"=w5272:errorcluster)
        n3831 = local read "Scan Range (V)\n(of steps)"() -> (w5270:dbl)
        n3832 = property on="Scan Range (V)\n(of steps)" class="DigNum (strict)"("Val(Sgnl)"=w5270) -> ()  [unwired: 2 in, 2 out]
      }
    }
    n3833 = disable-structure shown="Disabled" {
      disable-tunnel: [w4371 _] -> w4038
      disable-tunnel: w4037 -> [w4370 _]
      disable-tunnel: w4036 -> [w4368 _]
      disable-tunnel: w4035 -> [w4367 _]
      disable-tunnel: w4034 -> [w4366 _]
      disable-tunnel: w4033 -> [w4365 _]
      disable-tunnel: w4014 -> [w4364 _]
      frame Disabled {
        n3834 = case shown="True" "Sound ON" {
          tunnel: [w4372 w4417] -> w4371
          tunnel: w4370 -> [w4372 w4416]
          tunnel: w4368 -> [_ _]
          tunnel: w4364 -> [_ w4375]
          tunnel: w4367 -> [_ _]
          tunnel: w4366 -> [_ w4386]
          tunnel: w4365 -> [_ w4396]
          frame False {
          }
          frame True {
            n3835 = Index Array(array=w4375, index="Data channel to sound") -> (element=w4374:waveform(dbl))
            "Waveform Graph 2" <- w4374
            n3836 = Unbundle By Name(w4374) -> ("dt"=w4400:dbl, "Y"=w4398:dbl[])
            n3837 = Array Size(array=w4398) -> (size(s)=w4399:i32)
            "N data samples" <- w4399
            n3838 = for "Data time base" {
              N: w4399 -> [_]
              tunnel: [w4421] -> w4401 mode=indexing
              i -> [w4421]
            }
            n3839 = Multiply(x=w4400, y=w4401) -> (x*y=w4397:dbl[])
            n3840 = Compound Arithmetic op=MULTIPLY(6.283185307179586, "Carrier Frequency (Hz)", w4396) -> (w4413:dbl[])
            n3841 = call <vilib>:"Interpolate 1D.vi"("X is monotonic"=TRUE, "xi"=w4396, "X"=w4397, "Y"=w4398) -> ("yi"=w4394:dbl[])  [unwired: 5 in, 2 out]
            n3842 = Sine(x=w4413) -> (sin(x)=w4402:dbl[])
            n3843 = Add(x=w4394, y="Offset") -> (x+y=w4392:dbl[])
            n3844 = Multiply(x=w4392, y="mult x") -> (x*y=w4390:dbl[])
            n3845 = Add(x="Offset 2", y=w4390) -> (x+y=w4385:dbl[])
            n3846 = Compound Arithmetic op=MULTIPLY(6.283185307179586, "Carrier Frequency (Hz)", w4386, w4385) -> (w4377:dbl[])
            n3847 = for "Cumulative sum" {
              tunnel: [w4420] -> w4383 mode=indexing
              shift-right: [w4420] -> w4380
              shift-left: 0.0 -> [w4419]
              tunnel: w4377 -> [w4418] mode=indexing
              n3848 = Add(x=w4418, y=w4419) -> (x+y=w4420:dbl)
            }
            n3849 = feedback #46(0.0) -> (w4379:dbl)
            n3850 = Add(x=w4383, y=w4379) -> (x+y=w4382:dbl[])
            n3851 = Add(x=w4380, y=w4379) -> (x+y=w4378:dbl)
            n3852 = feedback-in #46(w4378) -> ()
            n3853 = Sine(x=w4382) -> (sin(x)=w4376:dbl[])
            n3854 = Select(t=w4402, s="tone or data", f=w4376) -> (s? t:f=w4408:dbl[])
            n3855 = Multiply(x=w4408, y="Volume") -> (x*y=w4406:dbl[])
            n3856 = Initialize Array(0.0 ("element"), "N initial buffer elements") -> (w4409:dbl[])
            n3857 = Multiply(x="N initial buffer elements", y=w4386) -> (x*y=→"Initial buffer time (s)":dbl)
            n3858 = Build Array (concatenate)(w4409, w4406) -> (w4411:dbl[])
            n3859 = First Call?() -> (First Call?: T/F=w4412:bool)
            n3860 = Select(t=w4411, s=w4412, f=w4406) -> (s? t:f=w4405:dbl[])
            n3861 = call-poly <vilib>:"Sound Output Write.vi"("data"=w4405, "task ID"=w4416) -> ("task ID out"=w4417:T42)  [unwired: 8 in, 1 out]
          }
        }
      }
      frame Enabled {
      }
    }
    n3862 = node-c288() -> ()  [unwired: 2 out]
  }
  n3863 = disable-structure shown="Disabled" {
    disable-tunnel: w10 -> [w5939 _]
    frame Disabled {
      n3864 = call <vilib>:"Sound Output Clear.vi"("task ID"=w5939) -> ()  [unwired: 10 in, 1 out]
    }
    frame Enabled {
    }
  }
  n3865 = node-c288(w56) -> ()  [unwired: 1 out]
  n3866 = node-c288(w64) -> ()  [unwired: 1 out]
  n3867 = flat-sequence {
    tunnel: w71 -> [w5943]
    tunnel: w72 -> [w5944]
    tunnel: [w5942] -> w70
    tunnel: [w5941] -> w69
    tunnel: w68 -> [_]
    tunnel: w66 -> [_]
    tunnel: w62 -> [_]
    tunnel: w70 -> [w5945]
    tunnel: w69 -> [w5946]
    frame #0 {
      w5940 = FALSE ("AI to FIFO")
      n3868 = xnode "Read/Write Control"("FPGA VI Reference In"=w5944, "error in"=w5943, "AI to FIFO"=w5940, "APD to FIFO"=w5940) -> ("FPGA VI Reference Out"=w5942:T24, "error out"=w5941:errorcluster)
    }
    frame #1 {
      n3869 = xnode "Close FPGA VI Reference"("FPGA VI Reference In"=w5945, "error in"=w5946) -> ("error out"=→"error out":errorcluster)
    }
  }
